vi "UHR-Fleezers Control (host) - Avogadro v3.vi"() -> ()   [LabVIEW 2014] (continued)
            n1858 = Concatenate Strings("irun" ("string"), "\r") -> (w2929:string)
            n1859 = VISA Write(VISA resource name=w2925, write buffer=w2929) -> ()  [unwired: 1 in, 3 out]
          }
          frame Enabled {
          }
        }
      }
      event "Stop Flow": Value Change {
        n1860 = event-data() -> ()  [unwired: 7 out]
        n1861 = disable-structure shown="Disabled" {
          disable-tunnel: w2931 -> [w2933 _]
          frame Disabled {
            w2932 = FALSE ("Stop Flow")
            n1862 = local write "Stop Flow"(w2932) -> ()
            n1863 = local write "Sample Channel\nFlow"(w2932) -> ()
            n1864 = Concatenate Strings("stop" ("string"), "\r") -> (w2935:string)
            n1865 = VISA Write(VISA resource name=w2933, write buffer=w2935) -> ()  [unwired: 1 in, 3 out]
          }
          frame Enabled {
          }
        }
      }
      event "Flow rate (uL/h)": Value Change {
        n1866 = event-data() -> ()  [unwired: 7 out]
        n1867 = disable-structure shown="Disabled" {
          disable-tunnel: w2937 -> [w2939 _]
          frame Disabled {
            n1868 = Number To Decimal String(number="Flow rate (uL/h)") -> (decimal integer string=w2943:string)  [unwired: 1 in]
            n1869 = Concatenate Strings("irate  " ("string"), w2943, " u/h" ("string"), "\r") -> (w2942:string)
            n1870 = VISA Write(VISA resource name=w2939, write buffer=w2942) -> ()  [unwired: 1 in, 3 out]
          }
          frame Enabled {
          }
        }
      }
      event "Flush Sample": Value Change {
        n1871 = event-data() -> ()  [unwired: 7 out]
        n1872 = disable-structure shown="Disabled" {
          disable-tunnel: ["Flush Sample" _] -> w2946
          disable-tunnel: w2945 -> [w2952 _]
          frame Disabled {
            n1873 = flat-sequence {
              tunnel: w2952 -> [w2993]
              tunnel: [w2973] -> w2956
              tunnel: [w2969] -> w2955
              tunnel: ["Volume (uL)"] -> w2951
              tunnel: ["Flush rate (uL/m)"] -> w2950
              tunnel: w2956 -> [w2997]
              tunnel: [w2997] -> w2954
              tunnel: w2955 -> [w2996]
              tunnel: w2954 -> [w3002]
              frame #0 {
                # "set paramaters (rate, volume) for flush, clear volume"
                n1874 = Number To Decimal String(number="Flush rate (uL/m)") -> (decimal integer string=w2989:string)  [unwired: 1 in]
                n1875 = Concatenate Strings("irate  " ("string"), w2989, " u/m" ("string"), "\r") -> (w2991:string)
                n1876 = VISA Write(VISA resource name=w2993, write buffer=w2991) -> (VISA resource name out=w2987:refnum<visa-resource-name>)  [unwired: 1 in, 2 out]
                n1877 = Reciprocal(x="Flush rate (uL/m)") -> (1/x=w2972:dbl)
                n1878 = Number To Decimal String(number="Volume (uL)") -> (decimal integer string=w2978:string)  [unwired: 1 in]
                n1879 = Multiply(x="Volume (uL)", y=w2972) -> (x*y=w2971:dbl)
                n1880 = Concatenate Strings("tvolume  " ("string"), w2978, " u" ("string"), "\r") -> (w2976:string)
                n1881 = Multiply(x=w2971, y=60000.0) -> (x*y=w2969:dbl)
                n1882 = VISA Write(VISA resource name=w2987, write buffer=w2976) -> (VISA resource name out=w2975:refnum<visa-resource-name>)  [unwired: 1 in, 2 out]
                n1883 = Concatenate Strings("cvolume" ("string"), "\r") -> (w2974:string)
                n1884 = VISA Write(VISA resource name=w2975, write buffer=w2974) -> (VISA resource name out=w2985:refnum<visa-resource-name>)  [unwired: 1 in, 2 out]
                n1885 = Concatenate Strings("irun" ("string"), "\r") -> (w2983:string)
                n1886 = VISA Write(VISA resource name=w2985, write buffer=w2983) -> (VISA resource name out=w2973:refnum<visa-resource-name>)  [unwired: 1 in, 2 out]
              }
              frame #1 {
                # "Have to wait until\nflow is done to reset\nrate"
                n1887 = Add(x=w2996, y=100.0) -> (x+y=w2995:dbl)
                n1888 = Wait (ms)(milliseconds to wait=w2995) -> ()  [unwired: 1 out]
              }
              frame #2 {
                # "reset flow rate to usual flow rate"
                n1889 = local read "Flow rate (uL/h)"() -> (w3008:dbl)
                n1890 = Number To Decimal String(number=w3008) -> (decimal integer string=w3006:string)  [unwired: 1 in]
                n1891 = Concatenate Strings("irate  " ("string"), w3006, " u/h" ("string"), "\r") -> (w3004:string)
                n1892 = VISA Write(VISA resource name=w3002, write buffer=w3004) -> (VISA resource name out=w2998:refnum<visa-resource-name>)  [unwired: 1 in, 2 out]
                n1893 = Concatenate Strings("cvolume" ("string"), "\r") -> (w2999:string)
                n1894 = VISA Write(VISA resource name=w2998, write buffer=w2999) -> ()  [unwired: 1 in, 3 out]
              }
            }
            n1895 = local read "Save Event Log?"() -> (w2948:bool)
            n1896 = local read "Saving..."() -> (w2947:bool)
            n1897 = And(x=w2948, y=w2947) -> (x .and. y?=w2949:bool)
            n1898 = case shown="True" w2949 {
              tunnel: w2951 -> [_ w2958]
              tunnel: w2950 -> [_ w2957]
              frame False {
              }
              frame True {
                n1899 = Number To Decimal String(number=w2958) -> (decimal integer string=w2962:string)  [unwired: 1 in]
                n1900 = Number To Decimal String(number=w2957) -> (decimal integer string=w2964:string)  [unwired: 1 in]
                n1901 = local read "log file ref"() -> (w2959:refnum<file>)
                n1902 = local read "Time (s)"() -> (w2960:dbl)
                n1903 = Concatenate Strings("pump 2 flushing ", w2962, " uL at ", w2964, " ul/min") -> (w2966:string)
                n1904 = call "write to event log.vi"("log file ref"=w2959, "time"=w2960, "input string"=w2966) -> ()  [unwired: 8 in]
              }
            }
          }
          frame Enabled {
          }
        }
      }
      event "Flush Pump 3": Value Change {
        n1905 = event-data() -> ()  [unwired: 7 out]
        n1906 = disable-structure shown="Disabled" {
          disable-tunnel: ["Flush Pump 3" _] -> w3010
          disable-tunnel: w3009 -> [w3016 _]
          frame Disabled {
            n1907 = flat-sequence {
              tunnel: w3016 -> [w3031]
              tunnel: ["Flush rate (uL/m) P3"] -> w3012
              tunnel: ["Volume (uL) P3"] -> w3011
              frame #0 {
                # "set paramaters (rate, volume) for flush, clear volume"
                n1908 = Number To Decimal String(number="Flush rate (uL/m) P3") -> (decimal integer string=w3051:string)  [unwired: 1 in]
                n1909 = local write "Inject Pump 3"(TRUE ("Inject Pump 3")) -> ()
                n1910 = Concatenate Strings("irate  " ("string"), w3051, " u/m" ("string"), "\r") -> (w3053:string)
                n1911 = VISA Write(VISA resource name=w3031, write buffer=w3053) -> (VISA resource name out=w3049:refnum<visa-resource-name>)  [unwired: 1 in, 2 out]
                n1912 = Reciprocal(x="Flush rate (uL/m) P3") -> (1/x=w3035:dbl)
                n1913 = Number To Decimal String(number="Volume (uL) P3") -> (decimal integer string=w3040:string)  [unwired: 1 in]
                n1914 = Multiply(x="Volume (uL) P3", y=w3035) -> (x*y=w3034:dbl)
                n1915 = Concatenate Strings("tvolume  " ("string"), w3040, " u" ("string"), "\r") -> (w3038:string)
                n1916 = Multiply(x=w3034, y=60.0) -> (x*y=→"HP3 Flush Time (s)":dbl)
                n1917 = VISA Write(VISA resource name=w3049, write buffer=w3038) -> (VISA resource name out=w3037:refnum<visa-resource-name>)  [unwired: 1 in, 2 out]
                n1918 = Concatenate Strings("cvolume" ("string"), "\r") -> (w3036:string)
                n1919 = VISA Write(VISA resource name=w3037, write buffer=w3036) -> (VISA resource name out=w3047:refnum<visa-resource-name>)  [unwired: 1 in, 2 out]
                n1920 = Concatenate Strings("irun" ("string"), "\r") -> (w3045:string)
                n1921 = VISA Write(VISA resource name=w3047, write buffer=w3045) -> ()  [unwired: 1 in, 3 out]
              }
              frame #1 {
                "Flushing P3" <- TRUE ("Flushing P3")
              }
            }
            n1922 = local read "Save Event Log?"() -> (w3014:bool)
            n1923 = local read "Saving..."() -> (w3015:bool)
            n1924 = And(x=w3014, y=w3015) -> (x .and. y?=w3013:bool)
            n1925 = case shown="True" w3013 {
              tunnel: w3012 -> [_ w3019]
              tunnel: w3011 -> [_ w3018]
              frame False {
              }
              frame True {
                n1926 = Number To Decimal String(number=w3018) -> (decimal integer string=w3023:string)  [unwired: 1 in]
                n1927 = Number To Decimal String(number=w3019) -> (decimal integer string=w3025:string)  [unwired: 1 in]
                n1928 = local read "log file ref"() -> (w3020:refnum<file>)
                n1929 = local read "Time (s)"() -> (w3021:dbl)
                n1930 = Concatenate Strings("pump 3 flushing ", w3023, " uL at ", w3025, " ul/min") -> (w3027:string)
                n1931 = call "write to event log.vi"("log file ref"=w3020, "time"=w3021, "input string"=w3027) -> ()  [unwired: 8 in]
              }
            }
          }
          frame Enabled {
          }
        }
      }
      event "Flush Pump 1": Value Change {
        n1932 = event-data() -> ()  [unwired: 7 out]
        n1933 = disable-structure shown="Disabled" {
          disable-tunnel: ["Flush Pump 1" _] -> w3057
          disable-tunnel: w3056 -> [w3063 _]
          frame Disabled {
            n1934 = flat-sequence {
              tunnel: [w3084] -> w3065
              tunnel: w3063 -> [w3079]
              tunnel: ["Volume (uL) P1"] -> w3059
              tunnel: ["Flush rate (uL/m) P1"] -> w3058
              tunnel: w3065 -> [_]
              frame #0 {
                # "set paramaters (rate, volume) for flush, clear volume"
                n1935 = local write "Inject Pump 1"(TRUE ("Inject Pump 1")) -> ()
                n1936 = Number To Decimal String(number="Flush rate (uL/m) P1") -> (decimal integer string=w3100:string)  [unwired: 1 in]
                n1937 = Concatenate Strings("irate  " ("string"), w3100, " u/m" ("string"), "\r") -> (w3102:string)
                n1938 = VISA Write(VISA resource name=w3079, write buffer=w3102) -> (VISA resource name out=w3098:refnum<visa-resource-name>)  [unwired: 1 in, 2 out]
                n1939 = Reciprocal(x="Flush rate (uL/m) P1") -> (1/x=w3083:dbl)
                n1940 = Number To Decimal String(number="Volume (uL) P1") -> (decimal integer string=w3089:string)  [unwired: 1 in]
                n1941 = Multiply(x="Volume (uL) P1", y=w3083) -> (x*y=w3082:dbl)
                n1942 = Concatenate Strings("tvolume  " ("string"), w3089, " u" ("string"), "\r") -> (w3087:string)
                n1943 = Multiply(x=w3082, y=60.0) -> (x*y=→"HP1 Flush Time (s)":dbl)
                n1944 = VISA Write(VISA resource name=w3098, write buffer=w3087) -> (VISA resource name out=w3086:refnum<visa-resource-name>)  [unwired: 1 in, 2 out]
                n1945 = Concatenate Strings("cvolume" ("string"), "\r") -> (w3085:string)
                n1946 = VISA Write(VISA resource name=w3086, write buffer=w3085) -> (VISA resource name out=w3096:refnum<visa-resource-name>)  [unwired: 1 in, 2 out]
                n1947 = Concatenate Strings("irun" ("string"), "\r") -> (w3094:string)
                n1948 = VISA Write(VISA resource name=w3096, write buffer=w3094) -> (VISA resource name out=w3084:refnum<visa-resource-name>)  [unwired: 1 in, 2 out]
              }
              frame #1 {
                "Flushing P1" <- TRUE ("Flushing P3")
              }
            }
            n1949 = local read "Saving..."() -> (w3060:bool)
            n1950 = local read "Save Event Log?"() -> (w3061:bool)
            n1951 = And(x=w3061, y=w3060) -> (x .and. y?=w3062:bool)
            n1952 = case shown="True" w3062 {
              tunnel: w3059 -> [_ w3068]
              tunnel: w3058 -> [_ w3067]
              frame False {
              }
              frame True {
                n1953 = Number To Decimal String(number=w3068) -> (decimal integer string=w3072:string)  [unwired: 1 in]
                n1954 = Number To Decimal String(number=w3067) -> (decimal integer string=w3070:string)  [unwired: 1 in]
                n1955 = local read "log file ref"() -> (w3074:refnum<file>)
                n1956 = local read "Time (s)"() -> (w3075:dbl)
                n1957 = Concatenate Strings("pump 1 flushing ", w3072, " uL at ", w3070, " ul/min") -> (w3066:string)
                n1958 = call "write to event log.vi"("log file ref"=w3074, "time"=w3075, "input string"=w3066) -> ()  [unwired: 8 in]
              }
            }
          }
          frame Enabled {
          }
        }
      }
      event "Clear Volume": Value Change {
        n1959 = event-data() -> ()  [unwired: 7 out]
        n1960 = disable-structure shown="Disabled" {
          disable-tunnel: ["Clear Volume" _] -> w3106
          disable-tunnel: w3105 -> [w3107 _]
          frame Disabled {
            n1961 = Concatenate Strings("cvolume" ("string"), "\r") -> (w3108:string)
            n1962 = VISA Write(VISA resource name=w3107, write buffer=w3108) -> ()  [unwired: 1 in, 3 out]
          }
          frame Enabled {
          }
        }
      }
      event "Clear Volume P3": Value Change {
        n1963 = event-data() -> ()  [unwired: 7 out]
        n1964 = disable-structure shown="Disabled" {
          disable-tunnel: w3112 -> [w3114 _]
          frame Disabled {
            n1965 = Concatenate Strings("cvolume" ("string"), "\r") -> (w3115:string)
            n1966 = VISA Write(VISA resource name=w3114, write buffer=w3115) -> ()  [unwired: 1 in, 3 out]
            n1967 = local write "Clear Volume P3"(FALSE ("Clear Volume P3")) -> ()
          }
          frame Enabled {
          }
        }
      }
      event "Clear Volume P1": Value Change {
        n1968 = event-data() -> ()  [unwired: 7 out]
        n1969 = disable-structure shown="Disabled" {
          disable-tunnel: w3118 -> [w3120 _]
          frame Disabled {
            n1970 = Concatenate Strings("cvolume" ("string"), "\r") -> (w3121:string)
            n1971 = local write "Clear Volume P1"(FALSE ("Clear Volume P1")) -> ()
            n1972 = VISA Write(VISA resource name=w3120, write buffer=w3121) -> ()  [unwired: 1 in, 3 out]
          }
          frame Enabled {
          }
        }
      }
      event "Display On P3": Value Change {
        n1973 = event-data() -> ()  [unwired: 7 out]
        n1974 = disable-structure shown="Disabled" {
          disable-tunnel: w3124 -> [w3125 _]
          frame Disabled {
            n1975 = Select(t="dim 100", s="Display On P3", f="dim 0") -> (s? t:f=w3128:string)
            n1976 = Concatenate Strings(w3128, "\r") -> (w3130:string)
            n1977 = VISA Write(VISA resource name=w3125, write buffer=w3130) -> ()  [unwired: 1 in, 3 out]
          }
          frame Enabled {
          }
        }
      }
      event "Display On P1": Value Change {
        n1978 = event-data() -> ()  [unwired: 7 out]
        n1979 = disable-structure shown="Disabled" {
          disable-tunnel: w3132 -> [w3133 _]
          frame Disabled {
            n1980 = Select(t="dim 100", s="Display On P1", f="dim 0") -> (s? t:f=w3136:string)
            n1981 = Concatenate Strings(w3136, "\r") -> (w3138:string)
            n1982 = VISA Write(VISA resource name=w3133, write buffer=w3138) -> ()  [unwired: 1 in, 3 out]
          }
          frame Enabled {
          }
        }
      }
      event "Retract Pump 3": Value Change {
        n1983 = event-data() -> ()  [unwired: 7 out]
        n1984 = disable-structure shown="Disabled" {
          disable-tunnel: w3140 -> [w3141 _]
          frame Disabled {
            n1985 = local write "Retract Pump 3"(FALSE ("Retract Pump 3")) -> ()
            n1986 = case shown="True" "Retract Pump 3" {
              tunnel: w3141 -> [_ w3144]
              frame False {
              }
              frame True {
                n1987 = Number To Decimal String(number="Retract Rate (uL/m)") -> (decimal integer string=w3162:string)  [unwired: 1 in]
                n1988 = Concatenate Strings("wrate  " ("string"), w3162, " u/m" ("string"), "\r") -> (w3164:string)
                n1989 = VISA Write(VISA resource name=w3144, write buffer=w3164) -> (VISA resource name out=w3155:refnum<visa-resource-name>)  [unwired: 1 in, 2 out]
                n1990 = Number To Decimal String(number="Retract Vol 3 (uL)") -> (decimal integer string=w3157:string)  [unwired: 1 in]
                n1991 = Concatenate Strings("tvolume  " ("string"), w3157, " u" ("string"), "\r") -> (w3154:string)
                n1992 = VISA Write(VISA resource name=w3155, write buffer=w3154) -> (VISA resource name out=w3150:refnum<visa-resource-name>)  [unwired: 1 in, 2 out]
                n1993 = Concatenate Strings("cvolume" ("string"), "\r") -> (w3151:string)
                n1994 = VISA Write(VISA resource name=w3150, write buffer=w3151) -> (VISA resource name out=w3145:refnum<visa-resource-name>)  [unwired: 1 in, 2 out]
                n1995 = Concatenate Strings("wrun" ("string"), "\r") -> (w3146:string)
                n1996 = VISA Write(VISA resource name=w3145, write buffer=w3146) -> ()  [unwired: 1 in, 3 out]
              }
            }
          }
          frame Enabled {
          }
        }
      }
      event "Retract Pump 1": Value Change {
        n1997 = event-data() -> ()  [unwired: 7 out]
        n1998 = disable-structure shown="Disabled" {
          disable-tunnel: w3166 -> [w3167 _]
          frame Disabled {
            n1999 = local write "Retract Pump 1"(FALSE ("Retract Pump 1")) -> ()
            n2000 = case shown="True" "Retract Pump 1" {
              tunnel: w3167 -> [_ w3172]
              frame False {
              }
              frame True {
                n2001 = local read "Retract Rate (uL/m)"() -> (w3170:dbl)
                n2002 = Number To Decimal String(number=w3170) -> (decimal integer string=w3188:string)  [unwired: 1 in]
                n2003 = Concatenate Strings("wrate  " ("string"), w3188, " u/m" ("string"), "\r") -> (w3190:string)
                n2004 = VISA Write(VISA resource name=w3172, write buffer=w3190) -> (VISA resource name out=w3182:refnum<visa-resource-name>)  [unwired: 1 in, 2 out]
                n2005 = Number To Decimal String(number="Retract Vol 1 (uL)") -> (decimal integer string=w3184:string)  [unwired: 1 in]
                n2006 = Concatenate Strings("tvolume  " ("string"), w3184, " u" ("string"), "\r") -> (w3181:string)
                n2007 = VISA Write(VISA resource name=w3182, write buffer=w3181) -> (VISA resource name out=w3178:refnum<visa-resource-name>)  [unwired: 1 in, 2 out]
                n2008 = Concatenate Strings("cvolume" ("string"), "\r") -> (w3179:string)
                n2009 = VISA Write(VISA resource name=w3178, write buffer=w3179) -> (VISA resource name out=w3173:refnum<visa-resource-name>)  [unwired: 1 in, 2 out]
                n2010 = Concatenate Strings("wrun" ("string"), "\r") -> (w3174:string)
                n2011 = VISA Write(VISA resource name=w3173, write buffer=w3174) -> ()  [unwired: 1 in, 3 out]
              }
            }
          }
          frame Enabled {
          }
        }
      }
      event "Flip Green Filter": Value Change {
        n2012 = event-data() -> ()  [unwired: 7 out]
        n2013 = Not(x="Flip Green Filter") -> (.not. x?=w3193:bool)
        n2014 = local write "Flip Green Filter"(w3193) -> ()
        n2015 = flat-sequence {
          tunnel: [w3202] -> w3198
          tunnel: [w3201] -> w3197
          tunnel: w3192 -> [w3200]
          tunnel: [w3205] -> w3196
          tunnel: w3198 -> [w3205]
          tunnel: [w3204] -> w3195
          tunnel: w3197 -> [w3204]
          tunnel: w3196 -> [w3209]
          tunnel: w3195 -> [w3208]
          tunnel: [w3207] -> w3199
          frame #0 {
            n2016 = xnode "Read/Write Control"("FPGA VI Reference In"=w3200, "Green Filter Flipper"=TRUE) -> ("FPGA VI Reference Out"=w3202:T41, "error out"=w3201:errorcluster)  [unwired: 1 in]
          }
          frame #1 {
            n2017 = Wait (ms)(milliseconds to wait=u32 100) -> ()  [unwired: 1 out]
          }
          frame #2 {
            n2018 = xnode "Read/Write Control"("FPGA VI Reference In"=w3209, "error in"=w3208, "Green Filter Flipper"=FALSE) -> ("error out"=w3207:errorcluster)  [unwired: 1 out]
          }
        }
      }
      event "Pump 1 contents", "Pump 3 contents": Value Change {
        n2019 = event-data() -> ()  [unwired: 7 out]
        n2020 = local read "Pump 1 contents"() -> (→"Pump 1 cont disp":string)
        n2021 = local read "Pump 3 contents"() -> (→"Pump 3 cont disp":string)
      }
      event "Reset Trap Pos. FB": Value Change {
        n2022 = event-data() -> ()  [unwired: 7 out]
        n2023 = xnode "Read/Write Control"("FPGA VI Reference In"=w3213, "Trap Pos. FB Reset"="Reset Trap Pos. FB") -> ()  [unwired: 1 in, 2 out]
      }
      event "Rem fb disp offset": Value Change {
        n2024 = event-data() -> ()  [unwired: 7 out]
        n2025 = local write "Rem fb disp offset"(FALSE ("Rem fb disp offset")) -> ()
        n2026 = local read "Mean Trap Positions (nm)"() -> (w3216:T6)
        n2027 = local read "FB Trap Pos Offset"() -> (w3218:dbl)
        n2028 = Unbundle By Name(w3216) -> ("T1 X"=w3215:dbl)
        n2029 = Subtract(x=w3218, y=w3215) -> (x-y=w3217:dbl)
        n2030 = local write "FB Trap Pos Offset"(w3217) -> ()
      }
      event "Threshold (nm)": Value Change {
        n2031 = event-data() -> ()  [unwired: 7 out]
        n2032 = flat-sequence {
          tunnel: [w3223] -> w3221
          tunnel: w3220 -> [w3222]
          tunnel: w3221 -> [w3234]
          frame #0 {
            n2033 = xnode "Read/Write Control"("FPGA VI Reference In"=w3222) -> ("FPGA VI Reference Out"=w3226:T41, "error out"=w3225:errorcluster, "FPGA TTrig Thresh"=w3227:i64)  [unwired: 1 in]
            n2034 = local read "Threshold stored (nm)"() -> (w3233:dbl)
            n2035 = local read "Threshold (nm)"() -> (w3223:dbl)
            n2036 = local read "AOM X Cal (nm/MHz)"() -> (w3231:dbl)
            n2037 = Subtract(x=w3223, y=w3233) -> (x-y=w3232:dbl)
            n2038 = Divide(x=w3232, y=w3231) -> (x/y=w3229:dbl)
            n2039 = call "IR AOM freq to word.vi"("Frequency In (MHz)"=w3229) -> ("Frequency Word Out (double)"=w3230:dbl)
            n2040 = To Quad Integer(1:w3230) -> (0:w3228:i64)
            n2041 = Add(x=w3227, y=w3228) -> (x+y=w3224:i64)
            n2042 = xnode "Read/Write Control"("FPGA VI Reference In"=w3226, "error in"=w3225, "FPGA TTrig Thresh"=w3224) -> ()  [unwired: 2 out]
          }
          frame #1 {
            "Threshold stored (nm)" <- w3234
          }
        }
      }
      event "FB Trig Integrate": Value Change {
        n2043 = event-data() -> ()  [unwired: 7 out]
        n2044 = local read "FB Trig Integrate"() -> (w3237:u32)
        n2045 = xnode "Read/Write Control"("FPGA VI Reference In"=w3235, "FB Trig Integrate"=w3237) -> ("error out"=w3236:errorcluster)  [unwired: 1 in, 1 out]
      }
      event "11": Value Change {
        n2046 = event-data() -> ()  [unwired: 7 out]
        n2047 = local read "11"() -> (w3238:bool)
        n2048 = case shown="True" w3238 {
          frame False {
          }
          frame True {
            n2049 = local read "Messages"() -> (w3240:string)
            n2050 = call "Update messages.vi"("Message to add"="You kicked it up to 11!", "Old message string"=w3240) -> ("New message string"=w3241:string)
            n2051 = call <vilib>:"Beep.vi"() -> ()  [unwired: 12 in]
            n2052 = local write "Messages"(w3241) -> ()
          }
        }
      }
      event "Trap Pos. FB ON": Value Change {
        w3248 = 6.0  # clock mult.
        w3247 = 49152000.0  # TCXO frequ.
        n2053 = event-data() -> ()  [unwired: 7 out]
        n2054 = xnode "Read/Write Control"("FPGA VI Reference In"=w3242) -> ("FPGA VI Reference Out"=w3244:T41, "BD1 Frequency Out 1"=w3245:u64)  [unwired: 1 in, 1 out]
        n2055 = To Double Precision Float(number=w3245) -> (double precision float=w3249:dbl)
        n2056 = Multiply(x=w3247, y=w3248) -> (x*y=w3250:dbl)
        n2057 = Multiply(x=w3249, y=w3250) -> (x*y=w3251:dbl)
        n2058 = Scale By Power Of 2(n=-48, x=w3251) -> (x*2^n=w3253:dbl)
        n2059 = Divide(x=w3253, y=1000000.0) -> (x/y=w3246:dbl)
        n2060 = flat-sequence {
          tunnel: w3244 -> [w3259]
          tunnel: [w3258] -> w3255
          tunnel: "Trap Pos. FB ON" -> [w3257]
          tunnel: w3245 -> [w3256]
          tunnel: w3255 -> [w3265]
          tunnel: "Trap Pos. FB ON" -> [w3264]
          tunnel: w3246 -> [w3267]
          tunnel: "Trap Pos. FB ON" -> [w3266]
          frame #0 {
            n2061 = case shown="False" w3257 {
              tunnel: w3259 -> [w3261 w3263]
              tunnel: [w3262 w3263] -> w3258
              tunnel: w3256 -> [w3260 _]
              frame False {
                n2062 = xnode "Read/Write Control"("FPGA VI Reference In"=w3261, "BD 1 Frequency 1"=w3260) -> ("FPGA VI Reference Out"=w3262:T41)  [unwired: 1 in, 1 out]
              }
              frame True {
              }
            }
          }
          frame #1 {
            n2063 = xnode "Read/Write Control"("FPGA VI Reference In"=w3265, "Force feedback"=w3264) -> ()  [unwired: 1 in, 2 out]
          }
          frame #2 {
            n2064 = case shown="False" w3266 {
              tunnel: w3267 -> [w3268 _]
              frame False {
                n2065 = property on="BD 1 Frequency 1 (MHz)" class="DigNum (strict)"("Val(Sgnl)"=w3268) -> ()  [unwired: 2 in, 2 out]
              }
              frame True {
              }
            }
          }
        }
      }
      event "Remove Action Offset": Value Change {
        n2066 = event-data() -> ()  [unwired: 7 out]
        n2067 = local write "Remove Action Offset"(FALSE ("Remove Action Offset")) -> ()
        n2068 = local read "Trap Pos. FB Mult Factor"() -> (w3274:i64)
        n2069 = local read "Trap Pos FB Action"() -> (w3272:i64)
        n2070 = local read "Trap Pos. FB Offset Factor"() -> (w3270:i64)
        n2071 = Multiply(x=w3274, y=w3272) -> (x*y=w3273:i64)
        n2072 = Add(x=w3273, y=w3270) -> (x+y=w3271:i64)
        n2073 = local write "Trap Pos. FB Offset Factor"(w3271) -> ()
        n2074 = xnode "Read/Write Control"("FPGA VI Reference In"=w3269, "Trap Pos. FB Offset Factor"=w3271) -> ()  [unwired: 1 in, 2 out]
      }
      event "Remove Unwinding Offset": Value Change {
        n2075 = event-data() -> ()  [unwired: 7 out]
        n2076 = local write "Remove Unwinding Offset"(FALSE ("Remove Action Offset")) -> ()
        n2077 = local read "Trap Pos. FB Mult Factor"() -> (w3288:i64)
        n2078 = local read "Trap Pos FB Action"() -> (w3286:i64)
        n2079 = local read "Trap Pos. FB Offset Factor"() -> (w3285:i64)
        n2080 = Multiply(x=w3288, y=w3286) -> (x*y=w3287:i64)
        n2081 = local read "Trap Pos. FB Mult Factor"() -> (w3284:i64)
        n2082 = Add(x=w3287, y=w3285) -> (x+y=w3278:i64)
        n2083 = Multiply(x=32768, y="factor") -> (x*y=w3281:dbl)
        n2084 = Multiply(x=w3281, y=w3284) -> (x*y=w3283:dbl)
        n2085 = Subtract(x=w3278, y=w3283) -> (x-y=w3282:dbl)
        n2086 = To Quad Integer(1:w3282) -> (0:w3277:i64)
        n2087 = xnode "Read/Write Control"("FPGA VI Reference In"=w3276, "Trap Pos. FB Offset Factor"=w3277) -> ()  [unwired: 1 in, 2 out]
        n2088 = local write "Trap Pos. FB Offset Factor"(w3277) -> ()
      }
      event "Trap Pos. FB Range", "Trap Pos. FB Gains", "Trap Pos. FB Mult Factor", "Trap Pos. FB Offset Factor", "Trap Pos FB Negate Action", "Trap Pos FB Monitor\nT1 or T2", "Differential FB?", "Negate Diff?": Value Change {
        n2089 = event-data() -> ()  [unwired: 7 out]
        n2090 = local read "Negate Diff?"() -> (w3293:bool)
        n2091 = xnode "Read/Write Control"("FPGA VI Reference In"=w3292, "Trap Pos. FB Gains"="Trap Pos. FB Gains", "Trap pos. FB Range"="Trap Pos. FB Range", "Trap Pos. FB Mult Factor"="Trap Pos. FB Mult Factor", "Trap Pos. FB Offset Factor"="Trap Pos. FB Offset Factor", "Trap Pos FB Negate Action"="Trap Pos FB Negate Action", "Trap Pos FB Monitor T1 or T2"="Trap Pos FB Monitor\nT1 or T2", "AI1 X Scale"="Trap Pos. AI1 X Pre-scale", "Negate Diff?"=w3293, "Diff FB Measurement?"="Differential FB?") -> ()  [unwired: 1 in, 2 out]
      }
      event "Trap Pos FB SP", "Trap Pos FB SP 2", "Use SP 2": Value Change {
        n2092 = event-data() -> ()  [unwired: 7 out]
        n2093 = Select(t="Trap Pos FB SP 2", s="Use SP 2", f="Trap Pos FB SP") -> (s? t:f=w3301:fxp<+/-,16,1>)
        n2094 = xnode "Read/Write Control"("FPGA VI Reference In"=w3300, "Trap Pos. FB SP"=w3301) -> ()  [unwired: 1 in, 2 out]
      }
      event "Offset SP2 from SP1": Value Change {
        n2095 = event-data() -> ()  [unwired: 7 out]
        n2096 = local read "Trap Pos FB SP"() -> (w3307:fxp<+/-,16,1>)
        n2097 = Add(x=w3307, y="SP2 Offset") -> (x+y=w3305:fxp<+/-,16,1>)
        n2098 = property on="Trap Pos FB SP 2" class="DigNum (strict)"("Val(Sgnl)"=w3305) -> ()  [unwired: 2 in, 2 out]
        n2099 = local write "Offset SP2 from SP1"(FALSE ("Offset SP2 from SP1")) -> ()
      }
      event "Set Reading to\nSetpoint": Value Change {
        # "This is the actual PID input signal"
        n2100 = event-data() -> ()  [unwired: 7 out]
        n2101 = local write "Set Reading to\nSetpoint"(FALSE ("Set SP to Reading")) -> ()
        n2102 = xnode "Read/Write Control"("FPGA VI Reference In"=w3311) -> ("FPGA VI Reference Out"=w3314:T41, "error out"=w3313:errorcluster, "Trap Pos FB Int-Norm Signal"=w3312:fxp<+/-,16,1>, "BD1 Frequency Out 1"=w3310:u64)  [unwired: 1 in]
        n2103 = local read "Differential FB?"() -> (w3315:bool)
        n2104 = case shown="False" w3315 {
          tunnel: [w3344 w3351] -> w3309
          tunnel: w3312 -> [w3342 w3351]
          frame False {
            n2105 = local read "Trap Pos FB Monitor\nT1 or T2"() -> (w3347:bool)
            n2106 = local read "Trap X AI1 (DMA)"() -> (w3350:T23)
            n2107 = Unbundle By Name(w3350) -> ("Set 1"=w3349:fxp<+/-,16,1>, "Set 2"=w3348:fxp<+/-,16,1>)
            n2108 = Select(t=w3349, s=w3347, f=w3348) -> (s? t:f=w3346:fxp<+/-,16,1>)
            n2109 = Not(x="Set SP Using...") -> (.not. x?=w3343:bool)
            n2110 = Select(t=w3342, s=w3343, f=w3346) -> (s? t:f=w3344:fxp<+/-,16,1>)
          }
          frame True {
          }
        }
        n2111 = disable-structure shown="Disabled" {
          disable-tunnel: _ -> [w3320 _]
          disable-tunnel: w3310 -> [w3319 _]
          disable-tunnel: w3309 -> [w3318 _]
          frame Disabled {
            n2112 = case shown="True" w3320 {
              tunnel: [w3321 w3323] -> w3317
              tunnel: w3318 -> [w3321 w3322]
              tunnel: w3319 -> [_ w3341]
              frame False {
              }
              frame True {
                w3339 = 6.0  # clock mult.
                w3340 = 49152000.0  # TCXO frequ.
                # "Added by Ronen - for the real time\nchange of the setpoint to accomodate \nchanges in the offset."
                n2113 = To Double Precision Float(number=w3341) -> (double precision float=w3338:dbl)
                n2114 = local read "BD 1 Frequency 2 (MHz)"() -> (w3331:dbl)
                n2115 = Multiply(x=w3340, y=w3339) -> (x*y=w3337:dbl)
                n2116 = Multiply(x=w3338, y=w3337) -> (x*y=w3336:dbl)
                n2117 = local read "Offset file step size"() -> (w3329:dbl)
                n2118 = Scale By Power Of 2(n=-48, x=w3336) -> (x*2^n=w3334:dbl)
                n2119 = Divide(x=w3334, y=1000000.0) -> (x/y=w3332:dbl)
                n2120 = Subtract(x=w3331, y=w3332) -> (x-y=w3330:dbl)
                n2121 = Divide(x=w3330, y=w3329) -> (x/y=w3328:dbl)
                n2122 = local read item#-1() -> (w3326)
                n2123 = To Long Integer(number=w3328) -> (32bit integer=w3327:i32)
                n2124 = Index Array(array=w3326, index=w3327) -> (element=w3325)
                n2125 = To Fixed-Point(number=w3325) -> (fixed-point=w3324:fxp<+/-,16,1>)  [unwired: 1 in]
                n2126 = Add(x=w3322, y=w3324) -> (x+y=w3323:fxp<+/-,17,2>)
              }
            }
            "Offset corrected setpoint" <- w3317
          }
          frame Enabled {
          }
        }
        n2127 = local write "Trap Pos FB SP"(w3309) -> ()
        n2128 = xnode "Read/Write Control"("FPGA VI Reference In"=w3314, "error in"=w3313, "Trap Pos. FB SP"=w3309) -> ()  [unwired: 2 out]
      }
      event "Trap Pos. FB Out Scale 2^n": Value Change {
        n2129 = event-data() -> ()  [unwired: 7 out]
        n2130 = Scale By Power Of 2(n="Trap Pos. FB Out Scale 2^n", x=ext 1.0) -> (x*2^n=w3352:ext)
        n2131 = property on="Trap Pos. FB Mult Factor" class="DigNum (strict)"("Val(Sgnl)"=w3352) -> ()  [unwired: 2 in, 2 out]
      }
      event "Trap Pos FB Int Count": Value Change {
        n2132 = event-data() -> ()  [unwired: 7 out]
        n2133 = xnode "Read/Write Control"("FPGA VI Reference In"=w3355, "Trap Pos FB Int Count"="Trap Pos FB Int Count") -> ()  [unwired: 1 in, 2 out]
      }
      event "Display Saved Data": Value Change {
        n2134 = event-data() -> ()  [unwired: 7 out]
        n2135 = case shown="\"Amp Current\"" "Display Saved Data" {
          frame "Bead Seperation", Default {
            n2136 = property on="Amp current" class="WFGraph (strict)"("Visible"=FALSE) -> ()  [unwired: 2 in, 2 out]
            n2137 = property on="Trap Delta Graph" class="WFGraph (strict)"("Visible"=TRUE) -> ()  [unwired: 2 in, 2 out]
            n2138 = property on="Saved trap pos" class="WFGraph (strict)"("Visible"=FALSE) -> ()  [unwired: 2 in, 2 out]
          }
          frame "Amp Current" {
            n2139 = property on="Saved trap pos" class="WFGraph (strict)"("Visible"=FALSE) -> ()  [unwired: 2 in, 2 out]
            n2140 = property on="Trap Delta Graph" class="WFGraph (strict)"("Visible"=FALSE) -> ()  [unwired: 2 in, 2 out]
            n2141 = property on="Amp current" class="WFGraph (strict)"("Visible"=TRUE) -> ()  [unwired: 2 in, 2 out]
          }
          frame "Trap Position" {
            n2142 = property on="Saved trap pos" class="WFGraph (strict)"("Visible"=TRUE) -> ()  [unwired: 2 in, 2 out]
            n2143 = property on="Trap Delta Graph" class="WFGraph (strict)"("Visible"=FALSE) -> ()  [unwired: 2 in, 2 out]
            n2144 = property on="Amp current" class="WFGraph (strict)"("Visible"=FALSE) -> ()  [unwired: 2 in, 2 out]
          }
        }
      }
      event "Calibration": Value Change {
        n2145 = event-data() -> ()  [unwired: 7 out]
        n2146 = local read "Calibration"() -> (w3381:u16)
        n2147 = Select(t="X" ("Label.Text"), s=TRUE, f="Y" ("Label.Text")) -> (s? t:f=w3378:string)
        n2148 = case shown="2" w3381 {
          tunnel: ["Position (V)" ("Label.Text") "Position (nm)" ("Label.Text") "Force (pN)" ("Label.Text")] -> w3375
          tunnel: [" (V)" ("Label.Text") " (nm)" ("Label.Text") " (pN)" ("Label.Text")] -> w3372
          frame 0, Default {
          }
          frame 1 {
          }
          frame 2 {
          }
        }
        n2149 = Concatenate Strings("T1 " ("Label.Text"), w3378) -> (w3374:string)
        n2150 = Concatenate Strings("T2 " ("Label.Text"), w3378) -> (w3373:string)
        n2151 = property on="Force" class="WFChart (strict)"("YScale.NameLbl.Text"=w3375) -> ()  [unwired: 2 in, 2 out]
        n2152 = Concatenate Strings("Mean" ("Label.Text"), w3372) -> (w3371:string)
        n2153 = Concatenate Strings(w3374, w3372) -> (w3370:string)
        n2154 = Concatenate Strings(w3373, w3372) -> (w3369:string)
        n2155 = Concatenate Strings("Difference" ("Label.Text"), w3372) -> (w3368:string)
        n2156 = property on="Mean" class="DigNum (strict)"("Caption.Text"=w3371) -> ()  [unwired: 2 in, 2 out]
        n2157 = property on="T1 X" class="DigNum (strict)"("Caption.Text"=w3370) -> ()  [unwired: 2 in, 2 out]
        n2158 = property on="T2 X" class="DigNum (strict)"("Caption.Text"=w3369) -> ()  [unwired: 2 in, 2 out]
        n2159 = property on="Difference" class="DigNum (strict)"("Caption.Text"=w3368) -> ()  [unwired: 2 in, 2 out]
      }
      event "Base N trap periods", "Period scale factor", "Trap osc amp (MHz)", "Cal sets to save", "# Samples/trap", "Total Counts (ticks)": Value Change {
        w3390 = 1.0
        w3396 = u32 0 ("y")
        # "scales 0 to 2pi"
        # "Create vector of trap offset (oscillation) values."
        # "Compute oscillation period as a multiple of the trap period. Should also fit nicely as a factor of the DMA period.\nCompare ticks for accurate commensurability check."
        # "Oscillation frequency needs to be commensurate\nwith the data save time."
        # "Be commensurate with total save time/100 (or so). That way you are guaranteed you can average spectra at least 100x."
        n2160 = event-data() -> ()  [unwired: 7 out]
        n2161 = local read "Total Counts (ticks)"() -> (w3412:u16)
        n2162 = To Unsigned Long Integer(number=w3412) -> (unsigned 32bit integer=w3422:u32)
        n2163 = Multiply "Base osc period (ticks)"(x=w3422, y="Base N trap periods") -> (x*y=w3413:u32)
        n2164 = local read "# Samples/trap"() -> (w3417:u32)
        n2165 = Multiply "Scaled osc period (ticks)"(x=w3413, y="Period scale factor") -> (x*y=w3414:dbl)
        n2166 = Multiply(x="Base N trap periods", y="Period scale factor") -> ()  [unwired: 1 out]
        n2167 = local read "Cal sets to save"() -> (w3418:u32)
        n2168 = To Unsigned Quad Integer(1:w3414) -> (0:w3404:u64)
        n2169 = for "vector 0 to N -1" {
          N: w3390 -> [_]
          tunnel: [w3439] -> w3410 mode=indexing
          i -> [w3439]
        }
        n2170 = Multiply "Ticks/DMA"(x=w3417, y=w3422) -> (x*y=w3421:u32)
        n2171 = Multiply "Scaled osc period (s)"(x=w3404, y=2.5e-08) -> (x*y=w3416:dbl)
        "Trap OSC Period (s)" <- w3416
        n2172 = Reciprocal(x=w3416) -> (1/x=→"A cal freq (Hz)":dbl)
        n2173 = Multiply(x=w3410, y=6.283185307179586) -> (x*y=w3425:dbl[])
        n2174 = Quotient & Remainder(x=w3421, y=w3404) -> (x-y*floor(x/y)=w3397:u64, floor(x/y)=→"N osc / DMA":u64)
        "DMA remainder" <- w3397
        n2175 = Multiply "Total trap ticks"(x=w3418, y=w3421) -> (x*y=w3405:u32)
        n2176 = Divide(x=w3425, y=w3390) -> (x/y=w3426:dbl[])
        n2177 = Sine(x=w3426) -> (sin(x)=w3427:dbl[])
        n2178 = Quotient & Remainder(x=w3405, y=100) -> (x-y*floor(x/y)=w3400:u32, floor(x/y)=w3420:u32)
        "Total save/100 remainder" <- w3400
        n2179 = Multiply "Single period osc vector"(x=w3427, y="Trap osc amp (MHz)") -> (x*y=w3403:dbl[])
        n2180 = Quotient & Remainder(x=w3420, y=w3404) -> (x-y*floor(x/y)=w3399:u64, floor(x/y)=→"N osc/ (total save/100)":u64)
        "(total save/100) /osc period remainder" <- w3399
        n2181 = Quotient & Remainder(x=w3405, y=w3404) -> (x-y*floor(x/y)=w3398:u64)  [unwired: 1 out]
        "N trap osc periods per save remainder" <- w3398
        n2182 = call "IR AOM freq to word - vec.vi"("Frequency In (double vec, MHz)"=w3403) -> ("Frequency Word Out"=w3402:dbl[])
        n2183 = To Quad Integer(1:w3402) -> (0:w3401:i64[])
        n2184 = disable-structure shown="Disabled" {
          disable-tunnel: w3409 -> [w3431 _]
          disable-tunnel: w3401 -> [w3429 _]
          frame Disabled {
            n2185 = xnode "Read/Write Control"("FPGA VI Reference In"=w3431) -> ("FPGA VI Reference Out"=w3430:T41)  [unwired: 3 in, 1 out]
            n2186 = flat-sequence {
              tunnel: w3429 -> [w3434]
              tunnel: w3430 -> [w3433]
              frame #0 {
                n2187 = for "Write data to fpga memory" {
                  tunnel: w3433 -> [w3436]
                  tunnel: w3434 -> [_] mode=indexing
                  (unwired) TRUE ("Ready Write")
                  n2188 = xnode "Read/Write Control"("FPGA VI Reference In"=w3436) -> ("FPGA VI Reference Out"=w3435:T41)  [unwired: 4 in, 1 out]
                  n2189 = while {
                    tunnel: w3435 -> [w3437]
                    stop <- _ continue-if-true
                    n2190 = xnode "Read/Write Control"("FPGA VI Reference In"=w3437) -> ()  [unwired: 1 in, 3 out]
                  }
                }
                "Writing waveform to fpga memory" <- TRUE ("Writing waveform to fpga memory")
              }
              frame #1 {
                n2191 = local write "Writing waveform to fpga memory"(FALSE ("Writing waveform to fpga memory")) -> ()
              }
            }
          }
          frame Enabled {
          }
        }
        n2192 = Equal?(x=w3399, y=w3396) -> (x = y?=w3394:bool)
        n2193 = Equal?(x=w3400, y=w3396) -> (x = y?=w3395:bool)
        n2194 = Equal?(x=w3397, y=w3396) -> (x = y?=w3392:bool)
        n2195 = Equal?(x=w3398, y=w3396) -> (x = y?=w3393:bool)
        n2196 = Compound Arithmetic op=AND(w3395, w3394, w3393, w3392) -> (→"Good freq?":bool)
      }
      event "Osc trap cont.", "Osc traps", "T1 Osc Enable", "T2 Osc Enable": Value Change {
        n2197 = event-data() -> ()  [unwired: 7 out]
        n2198 = disable-structure shown="Disabled" {
          disable-tunnel: w3440 -> [w3443 _]
          frame Disabled {
            n2199 = xnode "Read/Write Control"("FPGA VI Reference In"=w3443, "Trap 1 osc enable"="T1 Osc Enable", "Trap 2 osc enable"="T2 Osc Enable") -> ()  [unwired: 1 in, 2 out]
          }
          frame Enabled {
          }
        }
      }
      event "Pressure Pump Voltage (+/-10V)": Value Change {
        n2200 = event-data() -> ()  [unwired: 7 out]
        n2201 = disable-structure shown="Disabled" {
          disable-tunnel: w3444 -> [w3448 _]
          frame Disabled {
            n2202 = Divide(x="Pressure Pump Voltage (+/-10V)", y=10.0) -> (x/y=w3445:dbl)
            n2203 = Multiply(x=w3445, y=32767.0) -> (x*y=w3446:dbl)
            n2204 = xnode "Read/Write Control"("FPGA VI Reference In"=w3448, "Pressure Pump"=w3446) -> ()  [unwired: 1 in, 2 out]
          }
          frame Enabled {
          }
        }
      }
      event "Dynamic Force FB (ronen)": Value Change {
        # "Added by ronen - for feedback on trap position by changing the actual frequency and not the set frequency - for increasing the range of feedback."
        n2205 = event-data() -> ()  [unwired: 7 out]
        n2206 = xnode "Read/Write Control"("FPGA VI Reference In"=w3452, "Dynamic Force FB (Ronen)"="Dynamic Force FB (ronen)") -> ()  [unwired: 1 in, 2 out]
      }
      event "Read Setpoint Correction File": Value Change {
        n2207 = event-data() -> ()  [unwired: 7 out]
        n2208 = Open/Create/Replace File(file path (use dialog)="Setpoint Correction Offset File", operation (0:open)=T53."open", access (0:read/write)=enum16{"read/write", "read-only", "write-only"}."read-only") -> (refnum out=w3463:refnum<file>)  [unwired: 1 in, 4 out]
        n2209 = local write "Read Setpoint Correction File"(FALSE ("Read Setpoint Correction File")) -> ()
        n2210 = Deny Access(7:w3463) -> (3:w3462:refnum<file>)  [unwired: 1 in, 2 out]
        n2211 = Read from Binary File(5:0.0, 9:T54."big-endian, network order" ("byte order (0:big-endian, network order)"), 10:-1 ("count (1)"), 11:w3462) -> (2:w3453:dbl[], 3:w3461:refnum<file>)  [unwired: 1 in, 3 out]
        n2212 = Close File(refnum=w3461) -> ()  [unwired: 1 in, 2 out]
        n2213 = local read "Multiple-MCL offset?"() -> (w3455:bool)
        n2214 = local write "Raw offsets"(w3453) -> ()
        n2215 = case shown="True" w3455 {
          tunnel: w3453 -> [w3474 w3481]
          tunnel: [w3473 w3479] -> w3458
          tunnel: [w3472 w3478] -> w3457
          frame False {
            # "If not doing multiple offset, same calculation as before"
            n2216 = Decimate 1D Array(w3474) -> (w3473:dbl[], w3472:dbl[])
            n2217 = local read "Two Trap Offset Values"() -> (w3471:T32)
            n2218 = Bundle By Name(cluster=w3471, "Trap 1X offset"=w3473, "Trap 2X offset"=w3472) -> (w3470:T32)
            n2219 = local write "Two Trap Offset Values"(w3470) -> ()
          }
          frame True {
            w3476 = 0.0
            # "When doing multiple offset: separate data to different scans, make array of clusters of 1x,1y,2x,2y,3x,3y arrays"
            n2220 = local read "MCL offset scanning range (V)"() -> (w3482:T4)
            n2221 = local read "Offset file step size"() -> (w3480:dbl)
            n2222 = Build Array(w3476, w3476, w3476, w3476, w3476, w3476) -> (w3475:dbl[])
            n2223 = call "generate multiple MCL offset.vi"("Offset array"=w3481, "offset file step size"=w3480, "MCL offset scanning range (V)"=w3482, "Corrections"=w3475) -> ("B_X mean out"=w3478:dbl[], "A_X mean out"=w3479:dbl[], "Output array"=w3477:T31)
            n2224 = local write "Multi-MCL offset array"(w3477) -> ()
          }
        }
        n2225 = local read "B factor"() -> (w3454:dbl)
        n2226 = Multiply(x=w3457, y=w3454) -> (x*y=w3459:dbl[])
        n2227 = Subtract(x=w3458, y=w3459) -> (x-y=w3456:dbl[])
        n2228 = property on="Setpoint offset\ncorrection values" class="Arr (strict)"("Val(Sgnl)"=w3456) -> ()  [unwired: 2 in, 2 out]
      }
      event "B factor", "Setpoint offset\ncorrection values", "Target Force (pN)": Value Change {
        w3513 = 6.0  # clock mult.
        w3514 = 49152000.0  # TCXO frequ.
        n2229 = event-data() -> ()  [unwired: 7 out]
        n2230 = local read "B factor"() -> (w3515:dbl)
        n2231 = xnode "Read/Write Control"("FPGA VI Reference In"=w3516, "B factor"=w3515) -> ("BD1 Frequency Out 1"=w3506:u64)  [unwired: 1 in, 2 out]
        n2232 = To Double Precision Float(number=w3506) -> (double precision float=w3512:dbl)
        n2233 = local read "BD 1 Frequency 2 (MHz)"() -> (w3504:dbl)
        n2234 = Multiply(x=w3514, y=w3513) -> (x*y=w3511:dbl)
        n2235 = Multiply(x=w3512, y=w3511) -> (x*y=w3510:dbl)
        n2236 = Scale By Power Of 2(n=-48, x=w3510) -> (x*2^n=w3508:dbl)
        n2237 = Divide(x=w3508, y=1000000.0) -> (x/y=w3505:dbl)
        n2238 = Subtract(x=w3504, y=w3505) -> (x-y=w3492:dbl)
        n2239 = local read "Target Force (pN)"() -> (w3503:dbl)
        n2240 = local read "T1 calibration"() -> (w3501:T12)
        n2241 = local read "Offset file step size"() -> (w3491:dbl)
        n2242 = local read "Setpoint offset\ncorrection values"() -> (w3488:dbl[])
        n2243 = Unbundle By Name(w3501) -> ("alpha_x (nm/V)"=w3500:dbl, "kappa_x (pN/nm)"=w3499:dbl)
        n2244 = Multiply(x=w3503, y=2.0) -> (x*y=w3497:dbl)
        n2245 = Divide(x=w3492, y=w3491) -> (x/y=w3490:dbl)
        n2246 = local read "Negate Diff?"() -> (w3494:bool)
        n2247 = To Long Integer(number=w3490) -> (32bit integer=w3489:i32)
        n2248 = Multiply(x=w3500, y=w3499) -> (x*y=w3498:dbl)
        n2249 = Index Array(array=w3488, index=w3489) -> (element=w3486:dbl)
        n2250 = Divide(x=w3497, y=w3498) -> (x/y=w3493:dbl)
        n2251 = Select(t=1, s=w3494, f=-1) -> (s? t:f=w3487:i32)
        n2252 = Multiply(x=w3487, y=w3486) -> (x*y=w3485:dbl)
        n2253 = Add(x=w3493, y=w3485) -> (x+y=w3484:dbl)
        n2254 = To Fixed-Point(number=w3484) -> (fixed-point=w3483:fxp<+/-,16,1>)  [unwired: 1 in]
        n2255 = property on="Trap Pos FB SP" class="DigNum (strict)"("Val(Sgnl)"=w3483) -> ()  [unwired: 2 in, 2 out]
      }
      event "Trap 3 (ON/OFF)", "T3 Y (V)", "T3 X (V)": Value Change {
        n2256 = event-data() -> ()  [unwired: 7 out]
        n2257 = Multiply(x="T3 X (V)", y=32767.0) -> (x*y=w3534:dbl)
        n2258 = Multiply(x="T3 Y (V)", y=32767.0) -> (x*y=w3531:dbl)
        n2259 = Divide(x=w3534, y=10.0) -> (x/y=w3535:dbl)
        n2260 = Divide(x=w3531, y=10.0) -> (x/y=w3530:dbl)
        n2261 = To Word Integer(number=w3535) -> (16bit integer=w3524:i16)
        n2262 = To Word Integer(number=w3530) -> (16bit integer=w3525:i16)
        n2263 = case shown="False" "Trap 3 (ON/OFF)" {
          tunnel: [5.0 0.0] -> w3518
          frame False {
          }
          frame True {
          }
        }
        n2264 = Multiply(x=w3518, y=32767.0) -> (x*y=w3521:dbl)
        n2265 = Divide(x=w3521, y=10.0) -> (x/y=w3520:dbl)
        n2266 = To Word Integer(number=w3520) -> (16bit integer=w3517:i16)
        n2267 = xnode "Read/Write Control"("FPGA VI Reference In"=w3526, "Piezo Trap X (AO5)"=w3524, "Piezo Trap Y (AO4)"=w3525, "Piezo Trap ON/Off (AO3)"=w3517) -> ()  [unwired: 1 in, 2 out]
      }
      event "Cursor control.X", "Cursor control.Y": Value Change {
        # "If turning cursor control off, update the piezo controls"
        n2268 = event-data() -> ()  [unwired: 7 out]
        n2269 = xnode "Read/Write Control"("FPGA VI Reference In"=w3545) -> ("Piezo X out"=w3543:i16, "Piezo Y out"=w3539:i16)  [unwired: 1 in, 2 out]
        n2270 = local read "Cursor control"() -> (w3544:cluster{"X":bool, "Y":bool})
        n2271 = Unbundle By Name(w3544) -> ("X"=w3542:bool, "Y"=w3541:bool)
        n2272 = And(x=w3542, y=w3541) -> (x .and. y?=w3540:bool)
        n2273 = case shown="True" w3540 {
          tunnel: w3543 -> [w3550 _]
          tunnel: w3539 -> [w3548 _]
          frame False {
            w3547 = 3276.7
            n2274 = Divide(x=w3550, y=w3547) -> (x/y=w3549:dbl)
            n2275 = Divide(x=w3548, y=w3547) -> (x/y=w3546:dbl)
            n2276 = property on="T3 X (V)" class="DigNum (strict)"("Val(Sgnl)"=w3549) -> ()  [unwired: 2 in, 2 out]
            n2277 = property on="T3 Y (V)" class="DigNum (strict)"("Val(Sgnl)"=w3546) -> ()  [unwired: 2 in, 2 out]
          }
          frame True {
          }
        }
      }
      event "MCL offset scanning range (V)": Value Change {
        n2278 = event-data() -> ()  [unwired: 7 out]
        n2279 = local read "Multiple-MCL offset?"() -> (w3551:bool)
        n2280 = case shown="False" w3551 {
          frame False {
            # "Initialize the multi-MCL offset array"
            n2281 = local read "MCL offset scanning range (V)"() -> (w3557:T4)
            n2282 = local read "Offset file step size"() -> (w3553:dbl)
            n2283 = Divide(x=30.0, y=w3553) -> (x/y=w3554:dbl)
            n2284 = Initialize Array(0.0, w3554) -> (w3556:dbl[])
            n2285 = call "Make Trap3 position array.vi"("MCL offset scanning range (V)"=w3557) -> ("X Data points"=w3560:u64, "Y data points"=w3562:u64)  [unwired: 3 out]
            n2286 = Bundle(w3556, w3556, w3556, w3556, w3556, w3556) -> (w3559:T51)  [unwired: 1 in]
            n2287 = Multiply(x=w3562, y=w3560) -> (x*y=w3558:u64)
            n2288 = for {
              N: w3558 -> [_]
              tunnel: [w3564] -> w3561 mode=indexing
              tunnel: w3559 -> [w3564]
            }
            n2289 = Reshape Array(w3561, w3560, w3562) -> (w3563:T52)
            n2290 = local write "Multi-MCL offset array"(w3563) -> ()
          }
          frame True {
            n2291 = flat-sequence {
              frame #0 {
                n2292 = property on="Multiple-MCL offset?" class="Bool (strict)"("Val(Sgnl)"=FALSE) -> ()  [unwired: 2 in, 2 out]
              }
              frame #1 {
                n2293 = Wait (ms)(milliseconds to wait=200) -> ()  [unwired: 1 out]
              }
              frame #2 {
                # "Initialize the multi-MCL offset array"
                n2294 = local read "MCL offset scanning range (V)"() -> (w3572:T4)
                n2295 = local read "Offset file step size"() -> (w3568:dbl)
                n2296 = Divide(x=30.0, y=w3568) -> (x/y=w3569:dbl)
                n2297 = Initialize Array(0.0, w3569) -> (w3571:dbl[])
                n2298 = call "Make Trap3 position array.vi"("MCL offset scanning range (V)"=w3572) -> ("X Data points"=w3575:u64, "Y data points"=w3577:u64)  [unwired: 3 out]
                n2299 = Bundle(w3571, w3571, w3571, w3571, w3571, w3571) -> (w3574:T51)  [unwired: 1 in]
                n2300 = Multiply(x=w3577, y=w3575) -> (x*y=w3573:u64)
                n2301 = for {
                  N: w3573 -> [_]
                  tunnel: [w3579] -> w3576 mode=indexing
                  tunnel: w3574 -> [w3579]
                }
                n2302 = Reshape Array(w3576, w3575, w3577) -> (w3578:T52)
                n2303 = local write "Multi-MCL offset array"(w3578) -> ()
              }
              frame #3 {
                n2304 = Wait (ms)(milliseconds to wait=200) -> ()  [unwired: 1 out]
              }
              frame #4 {
                n2305 = property on="Multiple-MCL offset?" class="Bool (strict)"("Val(Sgnl)"=TRUE) -> ()  [unwired: 2 in, 2 out]
              }
            }
          }
        }
      }
      event "2D force calibration": Value Change {
        n2306 = event-data() -> ()  [unwired: 7 out]
        n2307 = local read "2D force calibration"() -> (w3582:u16)
        n2308 = case shown="1" w3582 {
          tunnel: ["Position (V)" ("Label.Text") "Position (nm)" ("Label.Text") "Force (pN)" ("Label.Text")] -> w3583
          frame 0, Default {
          }
          frame 1 {
          }
          frame 2 {
          }
        }
        n2309 = property on="2D forces" class="WFChart (strict)"("YScale.NameLbl.Text"=w3583) -> ()  [unwired: 2 in, 2 out]
      }
      event "T3 positioning test range (V)": Value Change {
        n2310 = event-data() -> ()  [unwired: 7 out]
        n2311 = flat-sequence {
          frame #0 {
            n2312 = local read "T3 positioning test range (V)"() -> (w3589:T10)
            n2313 = control-ref of="Correlations in X"() -> (w3588:refnum<vi>)
            n2314 = control-ref of="Correlations in Y"() -> (w3587:refnum<vi>)
            n2315 = Unbundle By Name(w3589) -> ("Xmin"=w3597:dbl, "increment"=w3602:dbl, "Ymin"=w3598:dbl, "Xmax"=w3599:dbl, "Ymax"=w3601:dbl)
            n2316 = Unbundle By Name(w3589) -> ("Xmin"=w3590:dbl, "increment"=w3595:dbl, "Ymin"=w3593:dbl, "Xmax"=w3591:dbl, "Ymax"=w3594:dbl)
            n2317 = Add(x=w3602, y=w3599) -> (x+y=w3600:dbl)
            n2318 = Add(x=w3602, y=w3601) -> (x+y=w3603:dbl)
            n2319 = Add(x=w3591, y=w3595) -> (x+y=w3592:dbl)
            n2320 = Add(x=w3594, y=w3595) -> (x+y=w3596:dbl)
            n2321 = property on="Property Node" class="IntGraph (strict)"(reference=w3587, "XScale.Minimum"=w3597, "XScale.Maximum"=w3600, "YScale.Minimum"=w3598, "YScale.Maximum"=w3603) -> ()  [unwired: 1 in, 2 out]
            n2322 = property on="Property Node" class="IntGraph (strict)"(reference=w3588, "XScale.Minimum"=w3590, "XScale.Maximum"=w3592, "YScale.Minimum"=w3593, "YScale.Maximum"=w3596) -> ()  [unwired: 1 in, 2 out]
          }
          frame #1 {
            n2323 = Wait (ms)(milliseconds to wait=50) -> ()  [unwired: 1 out]
          }
          frame #2 {
            n2324 = local read "T3 positioning test range (V)"() -> (w3607:T10)
            n2325 = control-ref of="Correlations in X"() -> (w3606:refnum<vi>)
            n2326 = control-ref of="Correlations in Y"() -> (w3605:refnum<vi>)
            n2327 = Unbundle By Name(w3607) -> ("Xmin"=w3611:dbl, "increment"=w3613:dbl, "Ymin"=w3612:dbl)
            n2328 = Unbundle By Name(w3607) -> ("Xmin"=w3608:dbl, "increment"=w3610:dbl, "Ymin"=w3609:dbl)
            n2329 = property on="Property Node" class="IntGraph (strict)"(reference=w3605, "XScale.Offset"=w3611, "XScale.Multiplier"=w3613, "YScale.Offset"=w3612, "YScale.Multiplier"=w3613) -> ()  [unwired: 1 in, 2 out]
            n2330 = property on="Property Node" class="IntGraph (strict)"(reference=w3606, "XScale.Offset"=w3608, "XScale.Multiplier"=w3610, "YScale.Offset"=w3609, "YScale.Multiplier"=w3610) -> ()  [unwired: 1 in, 2 out]
          }
        }
      }
      event "Scale intensities": Value Change {
        n2331 = event-data() -> ()  [unwired: 7 out]
        n2332 = local read "T2 calibration"() -> (w3621:T12)
        n2333 = local read "T1 calibration"() -> (w3614:T12)
        n2334 = local read "Setpoints (V)"() -> (w3629:cluster{"Set 1":dbl, "Set 2":dbl})
        n2335 = Unbundle By Name(w3614) -> ("kappa_x (pN/nm)"=w3625:dbl, "kappa_y (pN/nm)"=w3624:dbl)